vi "UHR-Fleezers Control (host) - 12.7b.vi"() -> ()   [LabVIEW 2012] (continued)
        n2060 = xnode "Read/Write Control"("FPGA VI Reference In"=w3017, "error in"=w3016, "Trap Pos. FB SP"=w3012) -> ()  [unwired: 2 out]
      }
      event "Offset SP2 from SP1": Value Change {
        n2061 = event-data() -> ()  [unwired: 7 out]
        n2062 = local read "Trap Pos FB SP"() -> (w3020:fxp<+/-,16,1>)
        n2063 = Add(x=w3020, y="SP2 Offset") -> (x+y=w3018:fxp<+/-,16,1>)
        n2064 = property on="Trap Pos FB SP 2" class="DigNum (strict)"("Val(Sgnl)"=w3018) -> ()  [unwired: 2 in, 2 out]
        n2065 = local write "Offset SP2 from SP1"(FALSE ("Offset SP2 from SP1")) -> ()
      }
      event "Set Reading to\nSetpoint": Value Change {
        # "This is the actual PID input signal"
        n2066 = event-data() -> ()  [unwired: 7 out]
        n2067 = local write "Set Reading to\nSetpoint"(FALSE ("Set SP to Reading")) -> ()
        n2068 = xnode "Read/Write Control"("FPGA VI Reference In"=w3026, "error in"=w3025) -> ("FPGA VI Reference Out"=w3024:T20, "error out"=w3023:errorcluster, "Trap Pos FB Int-Norm Signal"=w3022:fxp<+/-,16,1>)
        n2069 = local read "Differential FB?"() -> (w3027:bool)
        n2070 = case shown="False" w3027 {
          tunnel: [w3032 w3039] -> w3029
          tunnel: w3022 -> [w3030 w3039]
          frame False {
            n2071 = local read "Trap Pos FB Monitor\nT1 or T2"() -> (w3035:bool)
            n2072 = local read "Trap X AI1 (DMA)"() -> (w3038:T13)
            n2073 = Unbundle By Name(w3038) -> ("Set 1"=w3037:fxp<+/-,16,1>, "Set 2"=w3036:fxp<+/-,16,1>)
            n2074 = Select(t=w3037, s=w3035, f=w3036) -> (s? t:f=w3034:fxp<+/-,16,1>)
            n2075 = Not(x="Set SP Using...") -> (.not. x?=w3031:bool)
            n2076 = Select(t=w3030, s=w3031, f=w3034) -> (s? t:f=w3032:fxp<+/-,16,1>)
          }
          frame True {
          }
        }
        n2077 = xnode "Read/Write Control"("FPGA VI Reference In"=w3024, "error in"=w3023, "Trap Pos. FB SP"=w3029) -> ()  [unwired: 2 out]
        n2078 = local write "Trap Pos FB SP"(w3029) -> ()
      }
      event "Trap Pos. FB Out Scale 2^n": Value Change {
        n2079 = event-data() -> ()  [unwired: 7 out]
        n2080 = Scale By Power Of 2(n="Trap Pos. FB Out Scale 2^n", x=ext 1.0) -> (x*2^n=w3040:ext)
        n2081 = property on="Trap Pos. FB Mult Factor" class="DigNum (strict)"("Val(Sgnl)"=w3040) -> ()  [unwired: 2 in, 2 out]
      }
      event "Trap Pos FB Int Count": Value Change {
        n2082 = event-data() -> ()  [unwired: 7 out]
        n2083 = xnode "Read/Write Control"("FPGA VI Reference In"=w3045, "error in"=w3044, "Trap Pos FB Int Count"="Trap Pos FB Int Count") -> ()  [unwired: 2 out]
      }
      event "Trap pos": Value Change {
        n2084 = event-data() -> ()  [unwired: 7 out]
        n2085 = case shown="True" "Trap pos" {
          frame False {
            n2086 = property on="Trap Delta Graph" class="WFGraph (strict)"("Visible"=TRUE) -> ()  [unwired: 2 in, 2 out]
            n2087 = property on="Saved trap pos" class="WFGraph (strict)"("Visible"=FALSE) -> ()  [unwired: 2 in, 2 out]
          }
          frame True {
            n2088 = property on="Saved trap pos" class="WFGraph (strict)"("Visible"=TRUE) -> ()  [unwired: 2 in, 2 out]
            n2089 = property on="Trap Delta Graph" class="WFGraph (strict)"("Visible"=FALSE) -> ()  [unwired: 2 in, 2 out]
          }
        }
      }
    }
    "error out 2" <- w1867
    n2090 = node-c288() -> ()  [unwired: 2 out]
  }
  n2091 = timed-loop "Mouse control: trap position (AOM deflection), set confocal spot from image" {
    tunnel: [w3052] -> w213
    tunnel: w23 -> [w3051]
    timing: w135 -> [_]
    timing-out: [_] -> w134
    stop <- w3052 stop-if-true
    n2092 = node-c288() -> ()  [unwired: 2 out]
    n2093 = event shown="[0] \"Pane\": Mouse Down" {
      selector: _ -> [_ _]
      dyn-events: _ -> [_ _]
      timeout: _ -> [_ _]
      tunnel: w3051 -> [w3055 _]
      event Mouse Down {
        n2094 = event-data() -> ("Time"=w3057:u32, "Coords"=w3056:T7, "Button"=w3058:u16)  [unwired: 6 out]
        n2095 = case shown="3" w3058 {
          tunnel: w3057 -> [_ _ w3164]
          tunnel: w3056 -> [_ w3095 w3162]
          tunnel: w3055 -> [_ _ w3160]
          frame 0, Default {
          }
          frame 1 {
            n2096 = property on="APD 2" class="ImageControl"() -> ("Displayed Image Position"=w3065:cluster{"Left":i32, "Top":i32})  [unwired: 2 in, 2 out]
            n2097 = property on="APD 1" class="ImageControl"() -> ("Displayed Image Position"=w3094:cluster{"Left":i32, "Top":i32})  [unwired: 2 in, 2 out]
            n2098 = property on="Detection Laser X" class="ImageControl"() -> ("Displayed Image Position"=w3091:cluster{"Left":i32, "Top":i32})  [unwired: 2 in, 2 out]
            n2099 = property on="Detection Laser Y" class="ImageControl"() -> ("Displayed Image Position"=w3090:cluster{"Left":i32, "Top":i32})  [unwired: 2 in, 2 out]
            n2100 = property on="APD 2" class="ImageControl"() -> ("Displayed Image Size"=w3064:cluster{"Width":u32, "Height":u32})  [unwired: 2 in, 2 out]
            n2101 = property on="APD 1" class="ImageControl"() -> ("Displayed Image Size"=w3092:cluster{"Width":u32, "Height":u32})  [unwired: 2 in, 2 out]
            n2102 = property on="Detection Laser X" class="ImageControl"() -> ("Displayed Image Size"=w3093:cluster{"Width":u32, "Height":u32})  [unwired: 2 in, 2 out]
            n2103 = property on="Detection Laser Y" class="ImageControl"() -> ("Displayed Image Size"=w3089:cluster{"Width":u32, "Height":u32})  [unwired: 2 in, 2 out]
            n2104 = Unbundle By Name(w3064) -> ("Width"=w3061:u32, "Height"=w3060:u32)
            n2105 = Unbundle By Name(w3065) -> ("Left"=w3063:i32, "Top"=w3062:i32)
            n2106 = Unbundle By Name(w3092) -> ("Width"=w3086:u32, "Height"=w3085:u32)
            n2107 = Unbundle By Name(w3093) -> ("Width"=w3082:u32, "Height"=w3081:u32)
            n2108 = Unbundle By Name(w3089) -> ("Width"=w3078:u32, "Height"=w3077:u32)
            n2109 = Unbundle By Name(w3094) -> ("Left"=w3088:i32, "Top"=w3087:i32)
            n2110 = Unbundle By Name(w3091) -> ("Left"=w3084:i32, "Top"=w3083:i32)
            n2111 = Unbundle By Name(w3090) -> ("Left"=w3080:i32, "Top"=w3079:i32)
            n2112 = Bundle("Left"=w3063, "Top"=w3062, "Width"=w3061, "Height"=w3060) -> (w3059:T33)  [unwired: 1 in]
            n2113 = Bundle("Left"=w3088, "Top"=w3087, "Width"=w3086, "Height"=w3085) -> (w3076:T33)  [unwired: 1 in]
            n2114 = Bundle("Left"=w3084, "Top"=w3083, "Width"=w3082, "Height"=w3081) -> (w3075:T33)  [unwired: 1 in]
            n2115 = Bundle("Left"=w3080, "Top"=w3079, "Width"=w3078, "Height"=w3077) -> (w3074:T33)  [unwired: 1 in]
            n2116 = Build Cluster Array(w3059, w3076, w3075, w3074) -> (w3073:T34)
            n2117 = for {
              tunnel: w3095 -> [w3106]
              tunnel: w3073 -> [w3107] mode=indexing
              shift-right: [w3104] -> w3071
              shift-left: TRUE -> [w3105]
              shift-right: [w3103] -> w3069
              shift-left: _ -> [w3099]
              shift-right: [w3102] -> w3068
              shift-left: _ -> [w3098]
              shift-right: [w3101] -> w3067
              shift-left: _ -> [w3097]
              shift-right: [w3100] -> w3066
              shift-left: _ -> [w3096]
              n2118 = case shown="True" w3105 {
                selector: w3105 -> [w3112 _]
                tunnel: w3107 -> [_ w3121]
                tunnel: w3106 -> [_ w3119]
                tunnel: [w3112 w3117] -> w3104
                tunnel: [w3111 w3116] -> w3103
                tunnel: [w3110 w3115] -> w3102
                tunnel: [w3109 w3114] -> w3101
                tunnel: [w3108 w3113] -> w3100
                tunnel: w3099 -> [w3111 _]
                tunnel: w3098 -> [w3110 _]
                tunnel: w3097 -> [w3109 _]
                tunnel: w3096 -> [w3108 _]
                frame False {
                }
                frame True {
                  n2119 = Unbundle(w3121) -> (w3120:T33)
                  n2120 = call "isclickinwindow.vi"("Image Param"=w3120, "Point32"=w3119) -> ("4 Y"=w3113:i32, "3 Height"=w3114:i32, "2 X"=w3115:i32, "1 Width"=w3116:i32, "In image?"=w3118:bool)  [unwired: 1 in]
                  n2121 = Not(x=w3118) -> (.not. x?=w3117:bool)
                }
              }
            }
            n2122 = Not(x=w3071) -> (.not. x?=w3070:bool)
            n2123 = case shown="True" w3070 {
              tunnel: w3068 -> [_ w3135]
              tunnel: w3066 -> [_ w3134]
              tunnel: w3069 -> [_ w3133]
              tunnel: w3067 -> [_ w3132]
              frame False {
              }
              frame True {
                w3122 = FALSE ("Get Point")
                n2124 = local read "Scan lines (y)"() -> (w3137:u64)
                n2125 = disable-structure shown="Disabled" {
                  frame Disabled {
                  }
                  frame Enabled {
                  }
                }
                n2126 = local read "Actual MCL Inc (V)"() -> (w3131:dbl)
                n2127 = local read "Scan steps (MCL)"() -> (w3136:u64)
                n2128 = Divide "Y Pix/step"(x=w3132, y=w3137) -> (x/y=w3144:dbl)
                n2129 = Divide "Y V/pix"(x=w3131, y=w3144) -> (x/y=w3143:dbl)
                n2130 = Divide "Y half step offset"(x=w3131, y=2.0) -> (x/y=w3145:dbl)
                n2131 = Divide "X pix/step"(x=w3133, y=w3136) -> (x/y=w3142:dbl)
                n2132 = Negate(x=w3145) -> (-x=w3146:dbl)
                n2133 = local read "Initial Y"() -> (w3152:dbl)
                n2134 = Multiply(x=w3134, y=w3143) -> (x*y=w3153:dbl)
                n2135 = Divide "X half step offset"(x=w3131, y=2.0) -> (x/y=w3139:dbl)
                n2136 = Divide "X V/pix"(x=w3131, y=w3142) -> (x/y=w3141:dbl)
                n2137 = Multiply(x=w3131, y=w3136) -> (x*y=w3148:dbl)
                n2138 = Compound Arithmetic op=ADD(w3146, w3153, w3152) -> (w3123:dbl)
                "Pointer Y (V)" <- w3123
                n2139 = Multiply(x=w3141, y=w3135) -> (x*y=w3150:dbl)
                n2140 = Negate(x=w3139) -> (-x=w3138:dbl)
                n2141 = local read "Initial X"() -> (w3151:dbl)
                n2142 = Negate(x=w3150) -> (-x=w3149:dbl)
                n2143 = Compound Arithmetic op=ADD(w3138, w3148, w3151, w3149) -> (w3124:dbl)
                "Pointer X (V)" <- w3124
                n2144 = case shown="True" "Set High F Confocal Spot (X-Y)" {
                  tunnel: w3124 -> [_ w3154]
                  tunnel: w3123 -> [_ w3155]
                  frame False {
                  }
                  frame True {
                    "Confocal Y 2 (V)" <- w3155
                    "Confocal X 2 (V)" <- w3154
                  }
                }
                n2145 = Or(x="Set X Only", y="Set Confocal Spot (X-Y)") -> (x .or. y?=w3127:bool)
                n2146 = Or(x="Set Confocal Spot (X-Y)", y="Set Y Only") -> (x .or. y?=w3126:bool)
                n2147 = case shown="True" w3127 {
                  tunnel: w3124 -> [_ w3156]
                  frame False {
                  }
                  frame True {
                    n2148 = property on="AO2" class="Slide (strict)"("Val(Sgnl)"=w3156) -> ()  [unwired: 2 in, 2 out]
                    "Confocal X 1 (V)" <- w3156
                  }
                }
                n2149 = case shown="True" w3126 {
                  tunnel: w3123 -> [_ w3157]
                  frame False {
                  }
                  frame True {
                    n2150 = property on="AO1" class="Slide (strict)"("Val(Sgnl)"=w3157) -> ()  [unwired: 2 in, 2 out]
                    "Confocal Y 1 (V)" <- w3157
                  }
                }
                n2151 = local write "Set High F Confocal Spot (X-Y)"(w3122) -> ()
                n2152 = local write "Set Confocal Spot (X-Y)"(w3122) -> ()
                n2153 = local write "Set X Only"(w3122) -> ()
                n2154 = local write "Set Y Only"(w3122) -> ()
              }
            }
          }
          frame 3 {
            n2155 = local read "BD 2 Frequency 1 (MHz)"() -> (w3158:dbl)
            n2156 = local read "BD 1 Frequency 1 (MHz)"() -> (w3159:dbl)
            n2157 = local write "Manipulating Trap"(TRUE ("Manipulating Trap")) -> ()
            n2158 = local write "Coords"(T7 {"Horizontal"=0, "Vertical"=0} ("Coords")) -> ()
            n2159 = while {
              tunnel: w3164 -> [w3169]
              tunnel: w3162 -> [w3168]
              tunnel: w3160 -> [w3167]
              tunnel: w3159 -> [w3166]
              tunnel: w3158 -> [w3165]
              stop <- w3170 stop-if-true
              n2160 = event shown="[0] \"Pane\": Mouse Move" {
                selector: _ -> [_ _]
                dyn-events: _ -> [_ _]
                timeout: _ -> [_ _]
                tunnel: ["Force Manip Abort" w3234] -> w3170
                tunnel: w3169 -> [w3177 _]
                tunnel: w3168 -> [w3175 _]
                tunnel: w3167 -> [w3174 _]
                tunnel: w3166 -> [w3173 _]
                tunnel: w3165 -> [w3172 _]
                event Mouse Move {
                  n2161 = event-data() -> ("Time"=w3178:u32, "Coords"=w3179:T7)  [unwired: 3 out]
                  n2162 = Less?(x=w3178, y=w3177) -> (x < y?=w3176:bool)
                  n2163 = case "Makes sure old motion events prior to mouse click aren't used" shown="False" w3176 {
                    tunnel: w3179 -> [w3221 _]
                    tunnel: w3175 -> [w3222 _]
                    tunnel: w3174 -> [w3199 _]
                    tunnel: w3173 -> [w3195 _]
                    tunnel: w3172 -> [w3194 _]
                    frame False {
                      n2164 = Subtract(x=w3221, y=w3222) -> (x-y=w3220:T7)
                      "Coords" <- w3220
                      n2165 = local read "Y RF Frequency Limits (MHz)"() -> (w3180:T16)
                      n2166 = To Double Precision Float(number=w3220) -> (double precision float=w3219:cluster{"Horizontal":dbl, "Vertical":dbl})
                      n2167 = Multiply(x=cluster{"Horizontal":dbl, "Vertical":dbl} {"Horizontal"=-1.0, "Vertical"=1.0}, y="Manipulation Scaling") -> (x*y=w3215:cluster{"Horizontal":dbl, "Vertical":dbl})
                      n2168 = local read "X RF Frequency Limits (MHz)"() -> (w3181:T16)
                      n2169 = Multiply(x=w3219, y=w3215) -> (x*y=w3217:cluster{"Horizontal":dbl, "Vertical":dbl})
                      n2170 = Unbundle By Name(w3217) -> ("Horizontal"=w3212:dbl, "Vertical"=w3216:dbl)
                      n2171 = Unbundle By Name(w3180) -> ("Maximum"=w3183:dbl, "Minimum"=w3182:dbl)
                      n2172 = Boolean To (0,1)(Boolean="Manip. X?") -> (0, 1=w3210:i16)
                      n2173 = Boolean To (0,1)(Boolean="Manip. Y?") -> (0, 1=w3207:i16)
                      n2174 = local read "BD 1 Frequency 2 (MHz)"() -> (w3197:dbl)
                      n2175 = Multiply(x=w3216, y=w3207) -> (x*y=w3209:dbl)
                      n2176 = Multiply(x=w3210, y=w3212) -> (x*y=w3213:dbl)
                      n2177 = local read "BD 2 Frequency 2 (MHz)"() -> (w3196:dbl)
                      n2178 = Unbundle By Name(w3181) -> ("Maximum"=w3185:dbl, "Minimum"=w3184:dbl)
                      n2179 = Add(x=w3194, y=w3209) -> (x+y=w3187:dbl)
                      n2180 = Add(x=w3195, y=w3213) -> (x+y=w3189:dbl)
                      n2181 = In Range and Coerce(upper limit=w3185, x=w3189, lower limit=w3184) -> (coerced(x)=w3188:dbl)  [unwired: 1 out]
                      n2182 = In Range and Coerce(upper limit=w3183, x=w3187, lower limit=w3182) -> (coerced(x)=w3186:dbl)  [unwired: 1 out]
                      n2183 = Subtract(x=w3188, y=w3197) -> (x-y=w3206:dbl)
                      n2184 = Subtract(x=w3186, y=w3196) -> (x-y=w3205:dbl)
                      n2185 = Square(x=w3206) -> (x^2=w3204:dbl)
                      n2186 = Square(x=w3205) -> (x^2=w3203:dbl)
                      n2187 = Add(x=w3204, y=w3203) -> (x+y=w3202:dbl)
                      n2188 = Square Root(x=w3202) -> (sqrt(x)=w3198:dbl)
                      n2189 = In Range and Coerce(upper limit="Limit Max (MHz)", x=w3198, lower limit="Limit Min (MHz)") -> (In Range?=w3191:bool)  [unwired: 1 out]
                      n2190 = Not(x="Limits Enable") -> (.not. x?=w3190:bool)
                      n2191 = Or(x=w3191, y=w3190) -> (x .or. y?=w3192:bool)
                      n2192 = case shown="True" w3192 {
                        tunnel: w3199 -> [_ w3232]
                        tunnel: w3198 -> [_ w3223]
                        tunnel: w3188 -> [_ w3230]
                        tunnel: w3197 -> [_ w3229]
                        tunnel: w3186 -> [_ w3228]
                        tunnel: w3196 -> [_ w3227]
                        tunnel: w3181 -> [_ w3225]
                        tunnel: w3180 -> [_ w3224]
                        frame False {
                        }
                        frame True {
                          n2193 = local read "BD 1 Frequency 3 (MHz)"() -> (w3231:dbl)
                          n2194 = local read "BD 2 Frequency 3 (MHz)"() -> (w3226:dbl)
                          n2195 = local write "Trap Delta (MHz)"(w3223) -> ()
                          n2196 = call "set RF board frequency - interlace.vi"("Board 2 Frequency Limits"=w3224, "Board 1 Frequency Limits"=w3225, "FPGA VI Reference In"=w3232, "Board 2 Frequency 3 (MHz)"=w3226, "Board 1 Frequency 3 (MHz)"=w3231, "Board 2 Frequency 2 (MHz)"=w3227, "Board 2 Frequency 1 (MHz)"=w3228, "Board 1 Frequency 2 (MHz)"=w3229, "Board 1 Frequency 1  (MHz)"=w3230) -> ()  [unwired: 1 in, 2 out]
                          n2197 = local write "BD 2 Frequency 1 (MHz)"(w3228) -> ()
                          n2198 = local write "BD 1 Frequency 1 (MHz)"(w3230) -> ()
                        }
                      }
                    }
                    frame True {
                    }
                  }
                }
                event Mouse Up {
                  n2199 = event-data() -> ("Button"=w3233:u16)  [unwired: 8 out]
                  n2200 = case shown="3" w3233 {
                    tunnel: [FALSE TRUE] -> w3234
                    frame 0, Default {
                    }
                    frame 3 {
                      n2201 = local read "Trap Delta (MHz)"() -> (w3236:dbl)
                      n2202 = property on="Initial delta (MHz)" class="DigNum (strict)"("Val(Sgnl)"=w3236) -> ()  [unwired: 2 in, 2 out]
                      n2203 = local write "Manipulating Trap"(FALSE ("Manipulating Trap")) -> ()
                    }
                  }
                }
              }
            }
          }
        }
      }
      event Mouse Move {
        n2204 = event-data() -> ()  [unwired: 6 out]
      }
    }
    n2205 = local read "Stop All"() -> (w3052:bool)
    n2206 = node-c288() -> ()  [unwired: 2 out]
  }
  n2207 = timed-loop "Main data acquisition loop (get data, process data for display, and save data to disk)" {
    tunnel: w22 -> [w3548]
    tunnel: w94 -> [w3547]
    tunnel: [w3577] -> w298
    tunnel: [w3572] -> w296
    timing: w206 -> [_]
    timing-out: [_] -> w205
    tunnel: w111 -> [w3401]
    stop <- "Stop All" stop-if-true
    w3318 = "Initialize"
    # "Fluorescence data into FIFO for external control vi's\n(e.g., fluorescence triggering) - Duncan Nall"
    n2208 = node-c288() -> ()  [unwired: 2 out]
    n2209 = First Call?() -> (First Call?: T/F=w3353:bool)
    n2210 = Or(x="Reset", y=w3353) -> (x .or. y?=w3354:bool)
    n2211 = local read "Flushing P1"() -> (w3273:bool)
    n2212 = case "Reset data stream (manual reset or at begining of some rastering and imaging)" shown="True" w3354 {
      tunnel: w3548 -> [w4618 w4626]
      tunnel: w3547 -> [w4617 w4625]
      tunnel: [w4618 w4620] -> w3543
      tunnel: [w4617 w4619] -> w3542
      frame False {
      }
      frame True {
        w4623 = TRUE ("AI to FIFO")
        n2213 = local write "Overflow (data lost)"(FALSE ("Overflow (data lost)")) -> ()
        n2214 = call "reset FPGA DMA.vi"("error in"=w4625, "FPGA VI Reference In"=w4626) -> ("error out"=w4621:errorcluster, "FPGA VI Reference Out"=w4622:T20)
        n2215 = xnode "Read/Write Control"("FPGA VI Reference In"=w4622, "error in"=w4621, "AI to FIFO"=w4623, "APD to FIFO"=w4623) -> ("FPGA VI Reference Out"=w4620:T20, "error out"=w4619:errorcluster)
      }
    }
    n2216 = case shown="True" w3273 {
      frame False {
      }
      frame True {
        n2217 = local read "Flush rate (uL/m) P1"() -> (w3607:dbl)
        n2218 = local read "HP1 Flush Time (s)"() -> (w3616:dbl)
        n2219 = local read "DMA Update Period (s)"() -> (w3610:dbl)
        n2220 = Divide(x=w3607, y=60.0) -> (x/y=w3608:dbl)
        n2221 = Divide(x=w3616, y=w3610) -> (x/y=w3605:dbl)
        n2222 = feedback #1(0) -> (w3614:i32)
        n2223 = Increment(x=w3614) -> (x+1=w3604:i32)
        n2224 = Greater?(x=w3604, y=w3605) -> (0:w3613:bool)
        n2225 = Compound Arithmetic op=MULTIPLY(w3610, w3604, w3608) -> (→"P1 Flush Volume (uL)":dbl)
        n2226 = Divide(x=w3604, y=w3605) -> (x/y=→"P1 Flushing Bar":dbl)
        n2227 = case shown="True" w3613 {
          tunnel: w3604 -> [w3617 _]
          tunnel: [w3617 0] -> w3612
          frame False {
          }
          frame True {
            w3618 = FALSE ("Flushing P1")
            n2228 = local write "Inject Pump 1"(w3618) -> ()
            n2229 = local write "Flushing P1"(w3618) -> ()
            n2230 = property on="Clear Volume P1" class="Bool (strict)"("Val(Sgnl)"=TRUE ("Value (Signaling)")) -> ()  [unwired: 2 in, 2 out]
          }
        }
        n2231 = feedback-in #1(w3612) -> ()
      }
    }
    n2232 = Or(x="Start AOD Scan", y="Trap Raster Scan") -> (x .or. y?=w3499:bool)
    n2233 = case "Start AOM raster scan" shown="True" w3499 {
      tunnel: w3543 -> [w4468 w4478]
      tunnel: w3542 -> [w4467 w4477]
      tunnel: [w4468 w4471] -> w3541
      tunnel: [w4467 w4470] -> w3540
      frame False {
      }
      frame True {
        n2234 = case shown="True" "Restart DMA? (AOD)" {
          tunnel: [w4516 w4518] -> w4472
          tunnel: [w4515 w4517] -> w4473
          tunnel: w4478 -> [w4516 w4520]
          tunnel: w4477 -> [w4515 w4519]
          frame False {
          }
          frame True {
            n2235 = local write "Overflow (data lost)"(FALSE ("Overflow (data lost)")) -> ()
            n2236 = call "reset FPGA DMA.vi"("error in"=w4519, "FPGA VI Reference In"=w4520) -> ("error out"=w4517:errorcluster, "FPGA VI Reference Out"=w4518:T20)
          }
        }
        n2237 = local write "Trap Raster Scan"(FALSE ("Trap Raster Scan")) -> ()
        n2238 = case shown="True" "Move MCL Also?" {
          tunnel: w4473 -> [w4481 w4510]
          tunnel: w4472 -> [w4482 w4511]
          tunnel: [w4480 w4514] -> w4471
          tunnel: [w4479 w4513] -> w4470
          frame False {
            w4483 = TRUE ("AI to FIFO")
            n2239 = xnode "Read/Write Control"("FPGA VI Reference In"=w4482, "error in"=w4481, "AI to FIFO"=w4483, "APD to FIFO"=w4483, "Start scan"=w4483) -> ("FPGA VI Reference Out"=w4480:T20, "error out"=w4479:errorcluster)
          }
          frame True {
            w4507 = FALSE ("1D or 2D Scan?")
            w4512 = TRUE ("AI to FIFO")
            # "Count for MCL loop"
            # "N total cycles"
            # "N steps"
            # "V_int"
            n2240 = local read "Scan Range (nm)"() -> (w4489:dbl)
            n2241 = local read "Number of F/B Scans (AOD)"() -> (w4506:u16)
            n2242 = Sign(1:w4489) -> (0:w4488:dbl)
            n2243 = Compound Arithmetic op=MULTIPLY(w4489, "MCL Step Position Ratio", "MCL/AOM Scale Tweak") -> (w4493:dbl)
            n2244 = Negate(x=w4488) -> (-x=w4485:dbl)
            n2245 = Multiply(x=w4485, y="MCL Step Increment (V_int)") -> (x*y=w4487:dbl)
            n2246 = Divide(x=w4493, y="MCL X Cal (nm/V)") -> (x/y=w4499:dbl)
            n2247 = Multiply(x=32767.0 ("y"), y=w4499) -> (x*y=w4505:dbl)
            n2248 = local read "Total Counts (ticks)"() -> (w4490:u16)
            n2249 = local read "Cycles/step (AOD)"() -> (w4501:u64)
            n2250 = local read "Scan steps (AOD)"() -> (w4502:u64)
            n2251 = Divide(x=w4505, y=10.0) -> (x/y=w4498:dbl)
            n2252 = Divide(x=w4498, y="MCL Step Increment (V_int)") -> (x/y=w4496:dbl)
            n2253 = Absolute Value(x=w4496) -> (abs(x)=w4484:dbl)
            n2254 = Compound Arithmetic op=MULTIPLY(w4502, w4501, w4490) -> (w4497:u64)
            n2255 = local write "wait to reset values"(w4512) -> ()
            n2256 = local write "MCL Scanning"(w4512) -> ()
            n2257 = Divide(x=w4497, y=w4484) -> (x/y=w4494:dbl)
            "MCL Count" <- w4494
            n2258 = xnode "Read/Write Control"("FPGA VI Reference In"=w4511, "error in"=w4510, "Scan steps (MCL)"=w4484, "Number of scans (MCL)"=w4506, "Cycles per step (MCL)"=u64 1, "Scan freq.  increment (MCL)"=w4487, "1D or 2D Scan?"=w4507, "MCL Scan Axis"=w4507, "Cont. Scan (MCL)"=w4507, "MCL count"=w4494) -> ("FPGA VI Reference Out"=w4509:T20, "error out"=w4508:errorcluster)
            n2259 = xnode "Read/Write Control"("FPGA VI Reference In"=w4509, "error in"=w4508, "AI to FIFO"=w4512, "APD to FIFO"=w4512, "Start scan"=w4512, "Start scan (MCL)"=w4512) -> ("FPGA VI Reference Out"=w4514:T20, "error out"=w4513:errorcluster)
          }
        }
        "Raster Scanning..." <- TRUE ("Scanning...")
      }
    }
    n2260 = local read "Flushing P3"() -> (w3274:bool)
    n2261 = case "Keep track of when Harvard Pump 3 is done flushing" shown="True" w3274 {
      frame False {
      }
      frame True {
        n2262 = local read "Flush rate (uL/m) P3"() -> (w3624:dbl)
        n2263 = local read "DMA Update Period (s)"() -> (w3626:dbl)
        n2264 = local read "HP3 Flush Time (s)"() -> (w3633:dbl)
        n2265 = Divide(x=w3624, y=60.0) -> (x/y=w3622:dbl)
        n2266 = feedback #2(0) -> (w3631:i32)
        n2267 = Increment(x=w3631) -> (x+1=w3625:i32)
        n2268 = Divide(x=w3633, y=w3626) -> (x/y=w3627:dbl)
        n2269 = Greater?(x=w3625, y=w3627) -> (0:w3630:bool)
        n2270 = Compound Arithmetic op=MULTIPLY(w3626, w3625, w3622) -> (→"P3 Flush Volume (uL)":dbl)
        n2271 = case shown="True" w3630 {
          tunnel: w3625 -> [w3634 _]
          tunnel: [w3634 0] -> w3629
          frame False {
          }
          frame True {
            w3635 = FALSE ("Flushing P3")
            n2272 = local write "Inject Pump 3"(w3635) -> ()
            n2273 = local write "Flushing P3"(w3635) -> ()
            n2274 = property on="Clear Volume P3" class="Bool (strict)"("Val(Sgnl)"=TRUE ("Value (Signaling)")) -> ()  [unwired: 2 in, 2 out]
          }
        }
        n2275 = feedback-in #2(w3629) -> ()
        n2276 = Divide(x=w3625, y=w3627) -> (x/y=→"P3 Flushing Bar":dbl)
      }
    }
    n2277 = And(x="Save scans", y=w3499) -> (x .and. y?=w3539:bool)
    n2278 = Compound Arithmetic op=OR("Start MCL Scan", "Confocal Image", "Confocal Linescan") -> (w3497:bool)
    n2279 = And(x="Save Data (MCL)", y=w3497) -> (x .and. y?=w3538:bool)
    n2280 = case "Start MCL raster scan" shown="True" w3497 {
      tunnel: w3541 -> [w4080 w4096]
      tunnel: w3540 -> [w4079 w4095]
      tunnel: [w4080 w4091] -> w3400
      tunnel: [w4079 w4090] -> w3399
      tunnel: [FALSE w4089] -> w3524
      tunnel: "Start MCL Scan" -> [_ w4084]
      tunnel: "Confocal Image" -> [_ w4083]
      tunnel: "Confocal Linescan" -> [_ _]
      frame False {
      }
      frame True {
        w4089 = TRUE
        n2281 = case shown="True" "Restart DMA? (MCL)" {
          tunnel: [w4141 w4143] -> w4094
          tunnel: [w4140 w4142] -> w4093
          tunnel: w4096 -> [w4141 w4146]
          tunnel: w4095 -> [w4140 w4145]
          frame False {
          }
          frame True {
            n2282 = call "reset FPGA DMA.vi"("error in"=w4145, "FPGA VI Reference In"=w4146) -> ("error out"=w4142:errorcluster, "FPGA VI Reference Out"=w4143:T20)
            n2283 = local write "Overflow (data lost)"(FALSE ("Overflow (data lost)")) -> ()
          }
        }
        n2284 = case shown="False" w4084 {
          selector: w4084 -> [_ w4100]
          tunnel: w4083 -> [w4099 _]
          tunnel: [w4099 w4100] -> w4082
          frame False {
            n2285 = property on="2D or 1D Scan" class="Bool (strict)"("Val(Sgnl)"=w4099) -> ()  [unwired: 2 in, 2 out]
            n2286 = property on="Confocal Image" class="Bool (strict)"("Value"=FALSE ("Start Confocal Map")) -> ()  [unwired: 2 in, 2 out]
          }
          frame True {
          }
        }
        n2287 = local write "MCL Scanning"(w4089) -> ()
        n2288 = local read "AO1"() -> (w4086:dbl)
        n2289 = local read "AO2"() -> (w4085:dbl)
        n2290 = case shown="True" "Center Scan" {
          tunnel: w4094 -> [w4107 w4139]
          tunnel: w4093 -> [w4106 w4138]
          tunnel: [w4105 w4137] -> w4091
          tunnel: [w4104 w4136] -> w4090
          tunnel: [w4102 w4123] -> w4088
          tunnel: [w4101 w4122] -> w4087
          tunnel: w4086 -> [w4102 w4128]
          tunnel: w4085 -> [w4101 w4131]
          tunnel: w4082 -> [_ _]
          frame False {
            w4103 = TRUE ("AI to FIFO")
            n2291 = xnode "Read/Write Control"("FPGA VI Reference In"=w4107, "error in"=w4106, "AI to FIFO"=w4103, "APD to FIFO"=w4103, "Start scan (MCL)"=w4103) -> ("FPGA VI Reference Out"=w4105:T20, "error out"=w4104:errorcluster)
          }
          frame True {
            w4135 = TRUE ("AI to FIFO")
            n2292 = local read "Scan steps (MCL)"() -> (w4114:u64)
            n2293 = local read "Scan lines (y)"() -> (w4110:u64)
            n2294 = local read "Fast Scan Dir"() -> (w4121:bool)
            n2295 = local read "Actual MCL Inc (V)"() -> (w4111:dbl)
            n2296 = Decrement(x=w4110) -> (x-1=w4109:u64)
            n2297 = Decrement(x=w4114) -> (x-1=w4113:u64)
            n2298 = Multiply(x=w4111, y=w4109) -> (x*y=w4108:dbl)
            n2299 = Divide(x=w4108, y=2.0) -> (x/y=w4118:dbl)
            n2300 = Multiply(x=w4111, y=w4113) -> (x*y=w4112:dbl)
            n2301 = Divide(x=w4112, y=2.0) -> (x/y=w4117:dbl)
            n2302 = Select(t=w4117, s=w4121, f=w4118) -> (s? t:f=w4116:dbl)
            n2303 = Select(t=w4118, s=w4121, f=w4117) -> (s? t:f=w4120:dbl)
            n2304 = Subtract(x=w4128, y=w4120) -> (x-y=w4119:dbl)
            n2305 = Subtract(x=w4131, y=w4116) -> (x-y=w4115:dbl)
            n2306 = local read "2D or 1D Scan"() -> (w4133:bool)
            n2307 = Not(x=w4121) -> (.not. x?=w4127:bool)
            n2308 = Not(x=w4133) -> (.not. x?=w4129:bool)
            n2309 = And(x=w4121, y=w4129) -> (x .and. y?=w4130:bool)
            n2310 = And(x=w4129, y=w4127) -> (x .and. y?=w4132:bool)
            n2311 = Select(t=w4131, s=w4132, f=w4115) -> (s? t:f=w4122:dbl)
            n2312 = Select(t=w4128, s=w4130, f=w4119) -> (s? t:f=w4123:dbl)
            n2313 = call "Volt to I16.vi"("Voltage In"=w4123) -> ("I16 Voltage Out"=w4126:i16)
            n2314 = call "Volt to I16.vi"("Voltage In"=w4122) -> ("I16 Voltage Out"=w4125:i16)
            n2315 = xnode "Read/Write Control"("FPGA VI Reference In"=w4139, "error in"=w4138, "AI to FIFO"=w4135, "APD to FIFO"=w4135, "Start scan (MCL)"=w4135, "AO1"=w4126, "AO2"=w4125) -> ("FPGA VI Reference Out"=w4137:T20, "error out"=w4136:errorcluster)
          }
        }
        "Initial Y" <- w4088
        "Initial X" <- w4087
        n2316 = local write "Tab Control 6"(T3."Imaging" ("Tab Control 6")) -> ()
        "wait to reset values" <- w4089
      }
    }
    n2317 = local read "APD Elements/DMA read"() -> (w3241:u32)
    n2318 = local read "Trap AI Elements/DMA read"() -> (w3462:u32)
    n2319 = xnode "Get APD Data"("FPGA VI Reference In"=w3400, "error in"=w3399, "Number of Elements"=w3241, "Timeout (ms)"=-1) -> ("Data"=w3431:u32[], "Elements Remaining"=→"APD FIFO Elements Remaining":u32)  [unwired: 2 out]
    n2320 = local read "Trap Pos Elements/DMA read"() -> (w3396:u32)
    n2321 = xnode "Invoke Method"("FPGA VI Reference In"=w3400, "error in"=w3399, "Number of Elements"=w3396, "Timeout (ms)"=-1) -> ("Data"=w3360:u16[], "Elements Remaining"=→"Trap Pos FIFO El Remaining":u32)  [unwired: 2 out]
    n2322 = xnode "Get Trap Data"("FPGA VI Reference In"=w3400, "error in"=w3399, "Number of Elements"=w3462, "Timeout (ms)"=-1 ("Timeout")) -> ("FPGA VI Reference Out"=w3295:T20, "error out"=w3294:errorcluster, "Data"=w3361:i16[], "Elements Remaining"=w3585:u32)
    "FIFO El. Rem." <- w3585
    n2323 = local read "DMA Update Period (s)"() -> (w3463:dbl)
    n2324 = local read "Trap AI FIFO Depth"() -> (w3587:u32)
    n2325 = local read "Number of APDs"() -> (w3263:u8)
    n2326 = Decimate 1D Array(w3360) -> (w3357:u16[], w3359:u16[], w3358:u16[])
    n2327 = feedback #3(0.0) -> (w3389:dbl)
    n2328 = Add(x=w3463, y=w3389) -> (x+y=w3561:dbl)
    n2329 = feedback-in #3(w3561) -> ()
    n2330 = To Time Stamp(1:w3389) -> (0:w3388:timestamp)
    n2331 = Subtract(x=w3587, y=w3462) -> (x-y=w3586:u32)
    n2332 = To Unsigned Long Integer(number=w3357) -> (unsigned 32bit integer=w3356:u32[])
    n2333 = Join Numbers(hi=w3359, lo=w3358) -> ((hi.lo)=w3355:u32[])
    n2334 = Divide(x=w3585, y=w3586) -> (x/y=w3584:dbl)
    "Buffer Status" <- w3584
    n2335 = case "Deinterlace APD signals" shown="3, Default" w3263 {
      tunnel: [w3597 w3603] -> w3240
      tunnel: w3431 -> [w3598 w3602]
      tunnel: [w3596 w3601] -> w3239
      tunnel: [w3595 w3599] -> w3246
      frame 3, Default {
        n2336 = Decimate 1D Array "APD signals"(w3598) -> (w3597:u32[], w3596:u32[], w3595:u32[])
      }
      frame 2 {
        n2337 = Decimate 1D Array "APD signals"(w3602) -> (w3603:u32[], w3601:u32[])
        n2338 = Multiply(x=w3601, y=u32 0) -> (x*y=w3599:u32[])
      }
    }
    n2339 = Join Numbers(hi=w3356, lo=w3355) -> ((hi.lo)=w3349:u64[])
    n2340 = call "IR AOM word to freq - vec.vi"("Frequency Word In (double vec)"=w3349) -> ("Frequency Out"=w3395:dbl[])
    n2341 = Equal?(x=w3584, y=1.0) -> (x = y?=w3582:bool)
    n2342 = case "Alert buffer overflow" shown="True" w3582 {
      frame False {
      }
      frame True {
        n2343 = call <vilib>:"Beep.vi"() -> ()  [unwired: 3 in, 9 out]
        "Overflow (data lost)" <- TRUE ("Overflow (data lost)")
      }
    }
    n2344 = Decimate 1D Array(w3395) -> (w3394:dbl[], w3393:dbl[])
    n2345 = Build Array(w3394, w3393) -> (w3392:dbl[][])
    n2346 = Bundle(w3240, w3239, w3246) -> (w3244:cluster{u32[], u32[], u32[]})  [unwired: 1 in]
    n2347 = Build Array(w3240, w3239, w3246) -> (w3521:u32[][])
    n2348 = for {
      tunnel: w3240 -> [w3593] mode=indexing
      n2349 = call "Smart Buffer (DBL) 1.vi"("new element [write]"=w3593, "mode"=T21."write") -> ()  [unwired: 4 in, 6 out]
    }
    n2350 = local read "APD Integration Time (s)"() -> (w3256:dbl)
    n2351 = To Double Precision Float(number=w3521) -> (double precision float=w3522:dbl[][])
    n2352 = feedback #4 "APD3"(w3246) -> (w3262:u32[])
    n2353 = feedback #5 "APD2"(w3239) -> (w3418:u32[])
    n2354 = feedback #6 "APD1"(w3240) -> (w3520:u32[])
    n2355 = Build Array (concatenate)(w3418, w3239) -> (w3417:u32[])
    n2356 = Build Array (concatenate)(w3262, w3246) -> (w3261:u32[])
    n2357 = Build Array (concatenate)(w3520, w3240) -> (w3517:u32[])
    n2358 = for {
      tunnel: w3239 -> [w3592] mode=indexing
      n2359 = call "Smart Buffer (DBL) 2.vi"("new element [write]"=w3592, "mode"=T21."write") -> ()  [unwired: 4 in, 6 out]
    }
    n2360 = Array Size(array=w3517) -> (size(s)=w3514:i32)
    n2361 = Array Size(array=w3240) -> (size(s)=w3516:i32)
    n2362 = Multiply(x=w3516, y="APD Ave N") -> (x*y=w3515:dbl)
    n2363 = Greater?(x=w3514, y=w3515) -> (0:w3518:bool)
    n2364 = Bundle("APD 1", "APD 2", "APD 3") -> (w3554:cluster{string, string, string})  [unwired: 1 out]
    n2365 = local read "Trap Sets"() -> (w3461:u32)
    n2366 = case shown="True" w3518 {
      tunnel: w3517 -> [w3895 w3904]
      tunnel: [w3895 w3902] -> w3468
      tunnel: w3515 -> [_ w3897]
      tunnel: w3514 -> [_ w3903]
      tunnel: w3417 -> [w3894 w3901]
      tunnel: [w3894 w3900] -> w3415
      tunnel: w3261 -> [w3893 w3899]
      tunnel: [w3893 w3896] -> w3257
      frame False {
      }
      frame True {
        n2367 = Subtract(x=w3903, y=w3897) -> (x-y=w3898:dbl)
        n2368 = Array Subset "APD3"(array=w3899, index=w3898, length=w3897) -> (w3896:u32[])
        n2369 = Array Subset "APD2"(array=w3901, index=w3898, length=w3897) -> (w3900:u32[])
        n2370 = Array Subset "APD1"(array=w3904, index=w3898, length=w3897) -> (w3902:u32[])
      }
    }
    n2371 = feedback-in #4(w3257) -> ()
    n2372 = feedback-in #5(w3415) -> ()
    n2373 = feedback-in #6(w3468) -> ()
    n2374 = Cluster To Array(cluster=w3554) -> (array=w3551:string[])
    n2375 = for "APD" {
      tunnel: w3522 -> [w4151] mode=indexing
      tunnel: w3256 -> [w4158]
      tunnel: [w4154] -> w3419 mode=indexing
      tunnel: "APD Disp. Scale" -> [w4155]
      tunnel: w3551 -> [w4153] mode=indexing
      tunnel: "APD Disp. Downsample" -> [w4149]
      tunnel: [w4152] -> w3550
      workers-P: _ -> [_]
      tunnel: w3388 -> [w4148]
      n2376 = call "integrate 1D array interval - double.vi"("Ave N"=w4149, "Array In"=w4151) -> ("Array Out"=w4150:dbl[])  [unwired: 1 out]
      n2377 = Multiply(x=w4158, y=w4149) -> (x*y=w4152:dbl)
      n2378 = Divide(x=w4150, y=w4155) -> (x/y=w4156:dbl[])
      n2379 = Bundle By Name("t0"=w4148, "Y"=w4156, "dt"=w4152) -> (w4157:waveform(dbl))  [unwired: 1 out]
      n2380 = Set Waveform Attribute(5:w4153, 6:"NI_ChannelName" ("name"), 7:w4157) -> (3:w4154:waveform(dbl))  [unwired: 1 in, 2 out]
    }
    "APD Display Period (s)" <- w3550
    n2381 = Reciprocal(x=w3550) -> (1/x=→"APD Display Freq. (Hz)":dbl)
    n2382 = case "Deinterlace trap data, average down PSD" shown="2" w3461 {
      tunnel: w3361 -> [w4176 w4241]
      tunnel: [w4173 w4238] -> w3454
      tunnel: [w4176 w4240] -> w3352
      tunnel: "Detector Type" -> [w4175 w4236]
      tunnel: [w4174 w4239] -> w3453
      tunnel: [w4172 w4237] -> w3559
      frame 1, Default {
        n2383 = Divide(x=w4176, y=3276.7) -> (x/y=w4177:dbl[])
        n2384 = Decimate 1D Array(w4177) -> (w4186:dbl[], w4185:dbl[], w4184:dbl[], w4183:dbl[], w4182:dbl[], w4181:dbl[], w4180:dbl[], w4179:dbl[])
        n2385 = case shown="\"IR-QPD + PSD + FB-QPD position\"" w4175 {
          tunnel: w4186 -> [w4210 w4235]
          tunnel: w4185 -> [w4209 w4234]
          tunnel: w4184 -> [w4194 w4212]
          tunnel: w4183 -> [w4195 w4222]
          tunnel: w4182 -> [w4208 w4233]
          tunnel: w4181 -> [w4207 w4232]
          tunnel: w4180 -> [w4191 w4213]
          tunnel: w4179 -> [w4190 w4211]
          tunnel: [w4189 w4219] -> w4174
          tunnel: [w4188 w4218] -> w4173
          tunnel: [w4187 w4217] -> w4172
          frame "IR-QPD + PSD + FB-QPD", Default {
            w4187 = 0  # Channel pattern
            n2386 = Divide(x=w4210, y=w4195) -> (x/y=w4197:dbl[])
            n2387 = Divide(x=w4209, y=w4195) -> (x/y=w4196:dbl[])
            n2388 = Divide(x=w4208, y=w4191) -> (x/y=w4193:dbl[])
            n2389 = Divide(x=w4207, y=w4190) -> (x/y=w4192:dbl[])
            n2390 = Build Array(w4197, w4196, w4195, w4194, w4193, w4192, w4191, w4190) -> (w4188:dbl[][])
            n2391 = Bundle("T1 Y", "T1 X", "T1 Sum", "FB Sum", "PSD Y", "PSD X", "PSD Y Sum", "PSD X Sum") -> (w4206:T41)  [unwired: 1 out]
            n2392 = Cluster To Array(cluster=w4206) -> (array=w4189:string[])
          }
          frame "IR-QPD + PSD + FB-QPD position" {
            w4217 = 3  # Channel pattern
            n2393 = Negate(x=w4213) -> (-x=w4214:dbl[])
            n2394 = Divide(x=w4235, y=w4222) -> (x/y=w4224:dbl[])
            n2395 = Divide(x=w4234, y=w4222) -> (x/y=w4223:dbl[])
            n2396 = Divide(x=w4233, y=w4213) -> (x/y=w4221:dbl[])
            n2397 = Divide(x=w4232, y=w4214) -> (x/y=w4220:dbl[])
            n2398 = Build Array(w4224, w4223, w4222, w4211, w4212, w4221, w4220, w4213) -> (w4218:dbl[][])
            n2399 = Bundle("T1 Y", "T1 X", "T1 Sum", "FB X", "FB Sum", "PSD Y", "PSD X", "PSD Y Sum") -> (w4231:T41)  [unwired: 1 out]
            n2400 = Cluster To Array(cluster=w4231) -> (array=w4219:string[])
          }
        }
      }
      frame 2 {
        n2401 = case shown="\"IR-QPD + PSD + FB-QPD X position\"" w4236 {
          tunnel: w4241 -> [w4303 w4375 w4446]
          tunnel: [w4242 w4366 w4377] -> w4240
          tunnel: [w4269 w4357 w4424] -> w4239
          tunnel: [w4268 w4320 w4391] -> w4238
          tunnel: [w4262 w4355 w4422] -> w4237
          frame "IR-QPD + PSD + FB-QPD", Default {
            w4262 = 1  # Channel pattern
            # "time average x2 the 4th signal and the 4 psd signals (detection laser)"
            # "deinterlace 3 signals from qpd"
            n2402 = Decimate 1D Array(w4303) -> (w4302:i16[], w4301:i16[], w4267:i16[], w4300:i16[], w4290:i16[], w4288:i16[], w4287:i16[], w4285:i16[])
            n2403 = Decimate 1D Array(w4267) -> (w4266:i16[], w4265:i16[])
            n2404 = Decimate 1D Array(w4302) -> (w4299:i16[], w4271:i16[])
            n2405 = Decimate 1D Array(w4301) -> (w4298:i16[], w4296:i16[])
            n2406 = Decimate 1D Array(w4300) -> (w4297:i16[], w4295:i16[])
            n2407 = call "downsample 1D array - double.vi"("Ave N"=2.0, "Array In"=w4290) -> ("Array Out"=w4289:dbl[])  [unwired: 1 out]
            n2408 = call "downsample 1D array - double.vi"("Ave N"=2.0, "Array In"=w4288) -> ("Array Out"=w4270:dbl[])  [unwired: 1 out]
            n2409 = call "downsample 1D array - double.vi"("Ave N"=2.0, "Array In"=w4287) -> ("Array Out"=w4286:dbl[])  [unwired: 1 out]
            n2410 = call "downsample 1D array - double.vi"("Ave N"=2.0, "Array In"=w4285) -> ("Array Out"=w4284:dbl[])  [unwired: 1 out]
            n2411 = Interleave 1D Arrays(w4299, w4298, w4297, w4271, w4296, w4295, w4266, w4265, w4289, w4270, w4286, w4284) -> (w4283:dbl[])
            n2412 = Divide(x=w4283, y=3276.7) -> (x/y=w4282:dbl[])
            n2413 = Decimate 1D Array(w4282) -> (w4281:dbl[], w4280:dbl[], w4279:dbl[], w4278:dbl[], w4277:dbl[], w4276:dbl[], w4264:dbl[], w4263:dbl[], w4275:dbl[], w4274:dbl[], w4273:dbl[], w4272:dbl[])
            n2414 = Divide(x=w4281, y=w4279) -> (x/y=w4249:dbl[])
            n2415 = Divide(x=w4280, y=w4279) -> (x/y=w4248:dbl[])
            n2416 = Divide(x=w4278, y=w4276) -> (x/y=w4247:dbl[])
            n2417 = Divide(x=w4277, y=w4276) -> (x/y=w4246:dbl[])
            n2418 = Divide(x=w4275, y=w4273) -> (x/y=w4245:dbl[])
            n2419 = Divide(x=w4274, y=w4272) -> (x/y=w4244:dbl[])
            n2420 = Build Array(w4249, w4248, w4279, w4247, w4246, w4276, w4264, w4263, w4245, w4244, w4273, w4272) -> (w4268:dbl[][])
            n2421 = Bundle("T1 Y", "T1 X", "T1 Sum", "T2 Y", "T2 X", "T2 Sum", "T1 FB Sum", "T2 FB Sum", "PSD Y", "PSD X", "PSD Y Sum", "PSD X Sum") -> (w4250:T42)  [unwired: 1 out]
            n2422 = To Word Integer(number=w4283) -> (16bit integer=w4242:i16[])
            n2423 = Cluster To Array(cluster=w4250) -> (array=w4269:string[])
          }
          frame "IR-QPD + PSD + FB-QPD X position" {
            w4355 = 2  # Channel pattern
            # "time average x2 the 3 psd signals (detection laser)"
            # "deinterlace 3 signals from qpds"
            n2424 = Decimate 1D Array(w4375) -> (w4374:i16[], w4373:i16[], w4356:i16[], w4372:i16[], w4318:i16[], w4315:i16[], w4312:i16[], w4343:i16[])
            n2425 = Select(t=i16 -1, s="Flip X Sign", f=i16 1) -> (s? t:f=w4308:i16)
            n2426 = Multiply(x=w4373, y=w4308) -> (x*y=w4309:i16[])
            n2427 = Decimate 1D Array(w4356) -> (w4341:i16[], w4339:i16[])
            n2428 = Decimate 1D Array(w4374) -> (w4371:i16[], w4358:i16[])
            n2429 = Decimate 1D Array(w4309) -> (w4370:i16[], w4368:i16[])
            n2430 = Decimate 1D Array(w4372) -> (w4369:i16[], w4367:i16[])
            n2431 = Decimate 1D Array(w4343) -> (w4342:i16[], w4340:i16[])
            n2432 = call "downsample 1D array - I16.vi"("Ave N"=2.0, "Array In"=w4318) -> ("Array Out"=w4316:i16[])  [unwired: 1 in]
            n2433 = call "downsample 1D array - I16.vi"("Ave N"=2.0, "Array In"=w4312) -> ("Array Out"=w4310:i16[])  [unwired: 1 in]
            n2434 = call "downsample 1D array - I16.vi"("Ave N"=2.0, "Array In"=w4315) -> ("Array Out"=w4313:i16[])  [unwired: 1 in]
            n2435 = Interleave 1D Arrays(w4371, w4370, w4369, w4358, w4368, w4367, w4342, w4341, w4340, w4339, w4316, w4313, w4310) -> (w4366:i16[])
            n2436 = Divide(x=w4366, y=3276.7) -> (x/y=w4365:dbl[])
            n2437 = Decimate 1D Array(w4365) -> (w4364:dbl[], w4363:dbl[], w4362:dbl[], w4361:dbl[], w4360:dbl[], w4359:dbl[], w4331:dbl[], w4329:dbl[], w4328:dbl[], w4326:dbl[], w4325:dbl[], w4324:dbl[], w4321:dbl[])
            n2438 = Negate(x=w4321) -> (-x=w4319:dbl[])
            n2439 = Divide(x=w4325, y=w4321) -> (x/y=w4323:dbl[])
            n2440 = Divide(x=w4324, y=w4319) -> (x/y=w4322:dbl[])
            n2441 = Divide(x=w4364, y=w4362) -> (x/y=w4347:dbl[])
            n2442 = Divide(x=w4363, y=w4362) -> (x/y=w4346:dbl[])
            n2443 = Divide(x=w4361, y=w4359) -> (x/y=w4345:dbl[])
            n2444 = Divide(x=w4360, y=w4359) -> (x/y=w4344:dbl[])
            n2445 = Divide(x=w4331, y=w4329) -> (x/y=w4330:dbl[])
            n2446 = Divide(x=w4328, y=w4326) -> (x/y=w4327:dbl[])
            n2447 = Build Array(w4347, w4346, w4362, w4345, w4344, w4359, w4330, w4329, w4327, w4326, w4323, w4322, w4321) -> (w4320:dbl[][])
            n2448 = Bundle("T1 Y", "T1 X", "T1 Sum", "T2 Y", "T2 X", "T2 Sum", "T1 FB X", "T1 FB Sum", "T2 FB X", "T2 FB Sum", "PSD Y", "PSD X", "PSD Y Sum") -> (w4348:T43)  [unwired: 1 out]
            n2449 = Cluster To Array(cluster=w4348) -> (array=w4357:string[])
          }
          frame "IR-QPD + PSD + FB-QPD XY positions" {
            w4422 = 4  # Channel pattern
            # "time average x2 the 3 psd signals (detection laser)"
            # "deinterlace 3 signals from qpds"
            n2450 = Decimate 1D Array(w4446) -> (w4445:i16[], w4444:i16[], w4423:i16[], w4443:i16[], w4389:i16[], w4435:i16[], w4434:i16[], w4411:i16[])
            n2451 = Decimate 1D Array "Feedback Sum"(w4423) -> (w4407:i16[], w4405:i16[])
            n2452 = Decimate 1D Array "QPD Y"(w4445) -> (w4442:i16[], w4425:i16[])
            n2453 = Decimate 1D Array "QPD X"(w4444) -> (w4441:i16[], w4439:i16[])
            n2454 = Decimate 1D Array "Feedback Y"(w4389) -> (w4388:i16[], w4387:i16[])
            n2455 = Decimate 1D Array "QPD Sum"(w4443) -> (w4440:i16[], w4438:i16[])
            n2456 = Decimate 1D Array "Feedback X"(w4411) -> (w4408:i16[], w4406:i16[])
            n2457 = call "downsample 1D array - double.vi"("Ave N"=2.0, "Array In"=w4435) -> ("Array Out"=w4410:dbl[])  [unwired: 1 out]
            n2458 = call "downsample 1D array - double.vi"("Ave N"=2.0, "Array In"=w4434) -> ("Array Out"=w4409:dbl[])  [unwired: 1 out]
            n2459 = Interleave 1D Arrays(w4442, w4441, w4440, w4425, w4439, w4438, w4388, w4408, w4407, w4387, w4406, w4405, w4410, w4409) -> (w4433:dbl[])
            n2460 = Divide(x=w4433, y=3276.7) -> (x/y=w4432:dbl[])
            n2461 = Decimate 1D Array(w4432) -> (w4431:dbl[], w4430:dbl[], w4429:dbl[], w4428:dbl[], w4427:dbl[], w4426:dbl[], w4384:dbl[], w4398:dbl[], w4382:dbl[], w4383:dbl[], w4396:dbl[], w4380:dbl[], w4394:dbl[], w4392:dbl[])
            n2462 = Negate(x=w4392) -> (-x=w4390:dbl[])
            n2463 = Divide(x=w4394, y=w4390) -> (x/y=w4393:dbl[])
            n2464 = Divide(x=w4383, y=w4380) -> (x/y=w4379:dbl[])
            n2465 = Divide(x=w4384, y=w4382) -> (x/y=w4381:dbl[])
            n2466 = Divide(x=w4431, y=w4429) -> (x/y=w4415:dbl[])
            n2467 = Divide(x=w4430, y=w4429) -> (x/y=w4414:dbl[])
            n2468 = Divide(x=w4428, y=w4426) -> (x/y=w4413:dbl[])
            n2469 = Divide(x=w4427, y=w4426) -> (x/y=w4412:dbl[])
            n2470 = Divide(x=w4398, y=w4382) -> (x/y=w4397:dbl[])
            n2471 = Divide(x=w4396, y=w4380) -> (x/y=w4395:dbl[])
            n2472 = Build Array(w4415, w4414, w4429, w4413, w4412, w4426, w4381, w4397, w4382, w4379, w4395, w4380, w4393, w4392) -> (w4391:dbl[][])
            n2473 = Bundle("T1 Y", "T1 X", "T1 Sum", "T2 Y", "T2 X", "T2 Sum", "T1 FB Y", "T1 FB X", "T1 FB Sum", "T2 FB Y", "T2 FB X", "T2 FB Sum", "PSD X", "PSD Y Sum") -> (w4378:T44)  [unwired: 1 out]
            n2474 = To Word Integer(number=w4433) -> (16bit integer=w4377:i16[])
            n2475 = Cluster To Array(cluster=w4378) -> (array=w4424:string[])
          }
        }
      }
    }
    "AI labels" <- w3453
    n2476 = local read "APD Integration Time (s)"() -> (w3426:dbl)
    n2477 = Array Size(array=w3468) -> (size(s)=w3513:i32)
    n2478 = call <vilib>:"Std Deviation and Variance.vi"("X"=w3415) -> ("standard deviation"=w3414:dbl)  [unwired: 1 in, 2 out]
    n2479 = Add Array Elements(numeric array=w3415) -> (sum=w3416:u32)
    n2480 = Add Array Elements(numeric array=w3468) -> (sum=w3523:u32)
    n2481 = call <vilib>:"Std Deviation and Variance.vi"("X"=w3468) -> ("standard deviation"=w3467:dbl)  [unwired: 1 in, 2 out]
    n2482 = Divide(x=w3414, y=w3256) -> (x/y=w3411:dbl)
    "Rate sigma (Hz) 2" <- w3411
    n2483 = Multiply(x=w3256, y=w3513) -> (x*y=w3258:dbl)
    "Int. Time (s)" <- w3258
    n2484 = Divide(x=w3416, y=w3258) -> (x/y=w3412:dbl)
    "APD 2 Rate (Hz)" <- w3412
    n2485 = Multiply(x="APD Disp. Scale", y=w3419) -> (x*y=w3428:waveform(dbl)[])
    n2486 = Divide(x=w3523, y=w3258) -> (x/y=w3465:dbl)
    "APD 1 Rate (Hz)" <- w3465
    n2487 = Divide(x=w3467, y=w3256) -> (x/y=w3466:dbl)
    "Rate sigma (Hz)" <- w3466
    n2488 = Divide(x=w3411, y=w3412) -> (x/y=→"Sigma/Mean 2":dbl)
    n2489 = Multiply(x="APD Disp. Downsample", y=w3426) -> (x*y=w3424:dbl)
    n2490 = Divide(x=w3466, y=w3465) -> (x/y=→"Sigma/Mean":dbl)
    n2491 = Divide(x=w3428, y=w3424) -> (x/y=w3248:waveform(dbl)[])
    n2492 = Index Array(array=w3248, index=0) -> (element=w3408:waveform(dbl))
    n2493 = Index Array(array=w3248, index=1) -> (element=w3406:waveform(dbl))
    n2494 = Index Array(array=w3248, index=2) -> (element=w3250:waveform(dbl))
    n2495 = Subtract(x=w3408, y="APD 1 Offset") -> (x-y=w3404:waveform(dbl))
    n2496 = Subtract(x=w3406, y="APD 2 Offset") -> (x-y=w3403:waveform(dbl))
    n2497 = Subtract(x=w3250, y="APD 3 Offset") -> (x-y=w3247:waveform(dbl))
    n2498 = Add Array Elements(numeric array=w3257) -> (sum=w3260:u32)
    n2499 = call <vilib>:"Std Deviation and Variance.vi"("X"=w3257) -> ("standard deviation"=w3259:dbl)  [unwired: 1 in, 2 out]
    n2500 = Build Array(w3404, w3403, w3247) -> (→"APD Chart":waveform(dbl)[])
    n2501 = Divide(x=w3260, y=w3258) -> (x/y=w3254:dbl)
    "APD 3 Rate (Hz)" <- w3254
    n2502 = Divide(x=w3259, y=w3256) -> (x/y=w3255:dbl)
    "Rate sigma (Hz) 3" <- w3255
    n2503 = Divide(x=w3255, y=w3254) -> (x/y=→"Sigma/Mean 3":dbl)
    n2504 = local read "Data Period (s)"() -> (w3311:dbl)
    n2505 = local read "BD 1 Frequency 2 (MHz)"() -> (w3344:dbl)
    n2506 = local read "BD 1 Frequency 1 (MHz)"() -> (w3345:dbl)
    n2507 = Decimate 1D Array(w3352) -> (w3376:i16[], w3375:i16[], w3373:i16[], w3372:i16[])  [unwired: 9 out]
    n2508 = Multiply(x=w3311, y="Trap Pos. Disp. Downsample") -> (x*y=w3309:dbl)
    n2509 = Divide(x=w3376, y=w3375) -> (x/y=w3377:dbl[])
    n2510 = Divide(x=w3373, y=w3372) -> (x/y=w3374:dbl[])
    n2511 = local read "AOM X Cal (nm/MHz)"() -> (w3342:dbl)
    n2512 = Split 1D Array(array=w3377, index="N El. to Ave.") -> (second subarray=w3380:dbl[])  [unwired: 1 out]
    n2513 = Split 1D Array(array=w3374, index="N El. to Ave.") -> (second subarray=w3379:dbl[])  [unwired: 1 out]
    n2514 = Multiply(x=w3311, y="Trap Disp. Downsample") -> (x*y=w3390:dbl)
    "Display Period (s)" <- w3390
    n2515 = for "Trap AI" {
      tunnel: [w4171] -> w3555 mode=indexing
      tunnel: w3388 -> [w4162]
      tunnel: "Trap Disp. Downsample" -> [w4169]
      tunnel: w3454 -> [w4167] mode=indexing
      tunnel: w3311 -> [w4166]
      tunnel: w3453 -> [w4165] mode=indexing
      tunnel: [w4164] -> w3423 mode=indexing
      tunnel: w3390 -> [w4163]
      workers-P: _ -> [_]
      n2516 = Bundle By Name("Y"=w4167, "dt"=w4166) -> (w4168:waveform(dbl))  [unwired: 1 out]
      n2517 = Set Waveform Attribute(5:w4165, 6:"NI_ChannelName" ("name"), 7:w4168) -> (3:w4164:waveform(dbl))  [unwired: 1 in, 2 out]
      n2518 = call "downsample 1D array - double.vi"("Ave N"=w4169, "Array In"=w4167) -> ("Array Out"=w4170:dbl[])  [unwired: 1 out]
      n2519 = Bundle By Name(cluster=w4164, "t0"=w4162, "Y"=w4170, "dt"=w4163) -> (w4171:waveform(dbl))
    }
    n2520 = Bundle("BD 1 Frequency 1 (MHz)"=w3345, "BD 1 Frequency 2 (MHz)"=w3344) -> (w3346:T45)  [unwired: 1 out]
    n2521 = call-poly <vilib>:"Mean.vi"("X"=w3379) -> ("mean"=w3367:dbl)  [unwired: 1 out]
    n2522 = call-poly <vilib>:"Mean.vi"("X"=w3380) -> ("mean"=w3368:dbl)  [unwired: 1 out]
    n2523 = Reciprocal(x=w3390) -> (1/x=→"Trap Disp. Freq. (Hz)":dbl)
    n2524 = Cluster To Array(cluster=w3346) -> (array=w3343:dbl[])
    n2525 = local read "Trap X AI1 (DMA)"() -> (w3378:T13)
    n2526 = local read "Data points/scans (MCL)"() -> (w3533:dbl)
    n2527 = To Fixed-Point(number=w3367) -> (fixed-point=w3365:fxp<+/-,16,1>)  [unwired: 1 in]
    n2528 = To Fixed-Point(number=w3368) -> (fixed-point=w3366:fxp<+/-,16,1>)  [unwired: 1 in]
    n2529 = Bundle("Trap 1 Pos.", "Trap 2 Pos.") -> (w3387:cluster{string, string})  [unwired: 1 out]